vi "Dresden R2R Sputter 03.02.2018 IY24.vi"() -> ()   [LabVIEW 2009] (continued)
                                n27365 = local read "R Single DC Interval length"() -> (w32478:dbl)
                                n27366 = local read "Actual Length"() -> (w32482:dbl)
                                n27367 = Multiply(x=w32478, y=5.0) -> (x*y=w32476:dbl)
                                n27368 = Greater Or Equal?(x=w32482, y=w32476) -> (x >= y?=w32481:bool)
                                n27369 = local read "Semi"() -> (w32480:bool)
                                n27370 = Or(x=w32481, y=w32480) -> (x .or. y?=w32479:bool)
                                n27371 = Wait Until Next ms Multiple(millisecond multiple=u32 300) -> ()  [unwired: 1 out]
                                }
                                }
                                }
                                }
                                }
                                }
                                }
                                }
                                frame #1 {
                                }
                                }
                                }
                                frame #13 {
                                n27372 = local read "Semi"() -> (w32483:bool)
                                n27373 = case shown="False" w32483 {
                                frame #0 {
                                n27374 = local write "SDC1 13b"(TRUE ("SDC1 13b")) -> ()
                                n27375 = Wait (ms)(milliseconds to wait=u32 1000) -> ()  [unwired: 1 out]
                                }
                                frame #1 {
                                }
                                }
                                }
                                }
                                }
                                frame #1 {
                                }
                                }
                                }
                                frame #17 {
                                # "encoder info  add to other web selection"
                                n27376 = stacked-sequence {
                                frame #0 {
                                n27377 = local read "Semi"() -> (w32486:bool)
                                n27378 = case shown="False" w32486 {
                                frame #0 {
                                # "salinim hareketi"
                                n27379 = local read "R_Web_selection"() -> (w32487:enum32{"Web", "Other"})
                                n27380 = case shown="\"Other\"" w32487 {
                                frame #0 {
                                # "TC -ROLL"
                                }
                                frame #1 {
                                n27381 = disable-structure shown="Disabled" {
                                frame #0 {
                                # "OTHER"
                                n27382 = local read "Semi"() -> (w32488:bool)
                                n27383 = case shown="False" w32488 {
                                frame #0 {
                                n27384 = stacked-sequence {
                                frame #0 {
                                n27385 = local read "Semi"() -> (w32489:bool)
                                n27386 = case shown="False" w32489 {
                                frame #0 {
                                n27387 = stacked-sequence {
                                frame #0 {
                                n27388 = local read "Semi"() -> (w32490:bool)
                                n27389 = case shown="False" w32490 {
                                frame #0 {
                                n27390 = while {
                                i -> [w32493]
                                stop <- w32494 stop-if-true
                                n27391 = Greater?(x=w32493, y=300) -> (0:w32491:bool)
                                n27392 = case shown="True" w32491 {
                                frame #0 {
                                }
                                frame #1 {
                                n27393 = local write "Semi"(TRUE ("Semi")) -> ()
                                }
                                }
                                n27394 = local read "RC_13"() -> (w32497:bool)
                                n27395 = case shown="False" w32497 {
                                tunnel: [FALSE ("ch2_1") TRUE ("ch2_1")] -> w32496
                                frame #0 {
                                n27396 = local write "Routine_check_transfer"(TRUE ("ch2_1")) -> ()
                                n27397 = Wait Until Next ms Multiple(millisecond multiple=u32 1000) -> ()  [unwired: 1 out]
                                }
                                frame #1 {
                                }
                                }
                                n27398 = local read "Semi"() -> (w32495:bool)
                                n27399 = Or(x=w32496, y=w32495) -> (x .or. y?=w32494:bool)
                                }
                                }
                                frame #1 {
                                }
                                }
                                }
                                frame #1 {
                                n27400 = local read "Semi"() -> (w32503:bool)
                                n27401 = case shown="False" w32503 {
                                frame #0 {
                                n27402 = while {
                                i -> [w32510]
                                stop <- w32505 stop-if-true
                                n27403 = Greater?(x=w32510, y=100) -> (0:w32508:bool)
                                n27404 = case shown="True" w32508 {
                                frame #0 {
                                }
                                frame #1 {
                                n27405 = local write "Error Message"("Transfer process was cancelled.\nPlease check GV connections." ("Error Message")) -> ()
                                n27406 = local write "Semi"(TRUE ("Semi")) -> ()
                                }
                                }
                                n27407 = local read "Ch1_Trns_interlock_di"() -> (w32504:bool)
                                n27408 = case shown="False" w32504 {
                                tunnel: [w32512 TRUE] -> w32507
                                frame #0 {
                                n27409 = local read "Ch1_TGV_control_di"() -> (w32511:bool)
                                n27410 = case shown="False" w32511 {
                                tunnel: [FALSE TRUE] -> w32512
                                frame #0 {
                                n27411 = Wait Until Next ms Multiple(millisecond multiple=u32 50) -> ()  [unwired: 1 out]
                                n27412 = local write "Ch1_TGV_control_do"(TRUE ("Ch1_pet_cool_up_do")) -> ()
                                }
                                frame #1 {
                                }
                                }
                                }
                                frame #1 {
                                }
                                }
                                n27413 = local read "Semi"() -> (w32506:bool)
                                n27414 = Or(x=w32507, y=w32506) -> (x .or. y?=w32505:bool)
                                }
                                }
                                frame #1 {
                                }
                                }
                                }
                                frame #2 {
                                n27415 = local read "Semi"() -> (w32520:bool)
                                n27416 = case shown="False" w32520 {
                                frame #0 {
                                n27417 = while {
                                i -> [w32527]
                                stop <- w32522 stop-if-true
                                n27418 = Greater?(x=w32527, y=100) -> (0:w32525:bool)
                                n27419 = case shown="True" w32525 {
                                frame #0 {
                                }
                                frame #1 {
                                n27420 = local write "Error Message"("Transfer process was cancelled.\nPlease check GV connections." ("Error Message")) -> ()
                                n27421 = local write "Semi"(TRUE ("Semi")) -> ()
                                }
                                }
                                n27422 = local read "Ch2_Trns_interlock_di"() -> (w32521:bool)
                                n27423 = case shown="False" w32521 {
                                tunnel: [w32529 TRUE] -> w32524
                                frame #0 {
                                n27424 = local read "Ch2_TGV_control_di"() -> (w32528:bool)
                                n27425 = case shown="False" w32528 {
                                tunnel: [FALSE TRUE] -> w32529
                                frame #0 {
                                n27426 = Wait Until Next ms Multiple(millisecond multiple=u32 50) -> ()  [unwired: 1 out]
                                n27427 = local write "Ch2_TGV_control_do"(TRUE ("Ch1_pet_cool_up_do")) -> ()
                                }
                                frame #1 {
                                }
                                }
                                }
                                frame #1 {
                                }
                                }
                                n27428 = local read "Semi"() -> (w32523:bool)
                                n27429 = Or(x=w32524, y=w32523) -> (x .or. y?=w32522:bool)
                                }
                                }
                                frame #1 {
                                }
                                }
                                }
                                frame #3 {
                                n27430 = local read "Semi"() -> (w32537:bool)
                                n27431 = case shown="False" w32537 {
                                frame #0 {
                                n27432 = while {
                                i -> [w32544]
                                stop <- w32539 stop-if-true
                                n27433 = Greater?(x=w32544, y=100) -> (0:w32542:bool)
                                n27434 = case shown="True" w32542 {
                                frame #0 {
                                }
                                frame #1 {
                                n27435 = local write "Error Message"("Transfer process was cancelled.\nPlease check GV connections." ("Error Message")) -> ()
                                n27436 = local write "Semi"(TRUE ("Semi")) -> ()
                                }
                                }
                                n27437 = local read "Ch3_Trns_interlock_di"() -> (w32538:bool)
                                n27438 = case shown="False" w32538 {
                                tunnel: [w32546 TRUE] -> w32541
                                frame #0 {
                                n27439 = local read "Ch3_TGV_control_di"() -> (w32545:bool)
                                n27440 = case shown="False" w32545 {
                                tunnel: [FALSE TRUE] -> w32546
                                frame #0 {
                                n27441 = Wait Until Next ms Multiple(millisecond multiple=u32 50) -> ()  [unwired: 1 out]
                                n27442 = local write "Ch3_TGV_control_do"(TRUE ("Ch1_pet_cool_up_do")) -> ()
                                }
                                frame #1 {
                                }
                                }
                                }
                                frame #1 {
                                }
                                }
                                n27443 = local read "Semi"() -> (w32540:bool)
                                n27444 = Or(x=w32541, y=w32540) -> (x .or. y?=w32539:bool)
                                }
                                }
                                frame #1 {
                                }
                                }
                                }
                                frame #4 {
                                n27445 = local read "Semi"() -> (w32554:bool)
                                n27446 = case shown="False" w32554 {
                                frame #0 {
                                n27447 = while {
                                i -> [w32561]
                                stop <- w32556 stop-if-true
                                n27448 = Greater?(x=w32561, y=100) -> (0:w32559:bool)
                                n27449 = case shown="True" w32559 {
                                frame #0 {
                                }
                                frame #1 {
                                n27450 = local write "Error Message"("Transfer process was cancelled.\nPlease check GV connections." ("Error Message")) -> ()
                                n27451 = local write "Semi"(TRUE ("Semi")) -> ()
                                }
                                }
                                n27452 = local read "Ch3_Trns_interlock_di"() -> (w32555:bool)
                                n27453 = case shown="False" w32555 {
                                tunnel: [w32563 TRUE] -> w32558
                                frame #0 {
                                n27454 = local read "Ch3_TGV_control_di"() -> (w32562:bool)
                                n27455 = case shown="False" w32562 {
                                tunnel: [FALSE TRUE] -> w32563
                                frame #0 {
                                n27456 = Wait Until Next ms Multiple(millisecond multiple=u32 50) -> ()  [unwired: 1 out]
                                n27457 = local write "Ch3_TGV_control_do"(TRUE ("Ch1_pet_cool_up_do")) -> ()
                                }
                                frame #1 {
                                }
                                }
                                }
                                frame #1 {
                                }
                                }
                                n27458 = local read "Semi"() -> (w32557:bool)
                                n27459 = Or(x=w32558, y=w32557) -> (x .or. y?=w32556:bool)
                                }
                                }
                                frame #1 {
                                }
                                }
                                }
                                frame #5 {
                                n27460 = local read "Semi"() -> (w32571:bool)
                                n27461 = case shown="False" w32571 {
                                frame #0 {
                                n27462 = while {
                                i -> [w32574]
                                stop <- w32575 stop-if-true
                                n27463 = Greater?(x=w32574, y=50) -> (0:w32572:bool)
                                n27464 = case shown="True" w32572 {
                                frame #0 {
                                }
                                frame #1 {
                                n27465 = local write "Error Message"("Transfer process was\ncancelled.Please check right slow sensor." ("Error Message")) -> ()
                                n27466 = local write "Semi"(TRUE ("Semi")) -> ()
                                }
                                }
                                n27467 = local read "Cnt_Right_slow_di"() -> (w32578:bool)
                                n27468 = case shown="False" w32578 {
                                tunnel: [FALSE ("Ch1_pet_cool_up_do") TRUE ("Ch1_pet_cool_up_do")] -> w32577
                                frame #0 {
                                n27469 = local write "Cnt_Right_slow_do"(TRUE ("Ch1_pet_cool_up_do")) -> ()
                                n27470 = Wait Until Next ms Multiple(millisecond multiple=u32 200) -> ()  [unwired: 1 out]
                                }
                                frame #1 {
                                }
                                }
                                n27471 = local read "Semi"() -> (w32576:bool)
                                n27472 = Or(x=w32577, y=w32576) -> (x .or. y?=w32575:bool)
                                }
                                }
                                frame #1 {
                                }
                                }
                                }
                                frame #6 {
                                n27473 = local read "Semi"() -> (w32585:bool)
                                n27474 = case shown="False" w32585 {
                                frame #0 {
                                n27475 = while {
                                i -> [w32586]
                                stop <- w32590 stop-if-true
                                n27476 = Greater?(x=w32586, y=50) -> (0:w32588:bool)
                                n27477 = case shown="True" w32588 {
                                frame #0 {
                                }
                                frame #1 {
                                n27478 = local write "Error Message"("Transfer process was\ncancelled.Please check right limit sensor." ("Error Message")) -> ()
                                n27479 = local write "Semi"(TRUE ("Semi")) -> ()
                                }
                                }
                                n27480 = local read "Cnt_Right_limit_di"() -> (w32592:bool)
                                n27481 = case shown="False" w32592 {
                                tunnel: [FALSE ("Ch1_pet_cool_up_do") TRUE ("Ch1_pet_cool_up_do")] -> w32591
                                frame #0 {
                                n27482 = local write "Cnt_Right_limit_do"(TRUE ("Ch1_pet_cool_up_do")) -> ()
                                n27483 = Wait Until Next ms Multiple(millisecond multiple=u32 200) -> ()  [unwired: 1 out]
                                }
                                frame #1 {
                                }
                                }
                                n27484 = local read "Semi"() -> (w32589:bool)
                                n27485 = Or(x=w32591, y=w32589) -> (x .or. y?=w32590:bool)
                                }
                                }
                                frame #1 {
                                }
                                }
                                }
                                frame #7 {
                                n27486 = local read "Semi"() -> (w32599:bool)
                                n27487 = case shown="False" w32599 {
                                frame #0 {
                                n27488 = while {
                                i -> [w32602]
                                stop <- w32603 stop-if-true
                                n27489 = Greater?(x=w32602, y=50) -> (0:w32600:bool)
                                n27490 = case shown="True" w32600 {
                                frame #0 {
                                }
                                frame #1 {
                                n27491 = local write "Error Message"("Transfer process was\ncancelled.Please check left slow sensor." ("Error Message")) -> ()
                                n27492 = local write "Semi"(TRUE ("Semi")) -> ()
                                }
                                }
                                n27493 = local read "Cnt_Left_slow_di"() -> (w32606:bool)
                                n27494 = case shown="False" w32606 {
                                tunnel: [FALSE ("Ch1_pet_cool_up_do") TRUE ("Ch1_pet_cool_up_do")] -> w32605
                                frame #0 {
                                n27495 = local write "Cnt_Left_slow_do"(TRUE ("Ch1_pet_cool_up_do")) -> ()
                                n27496 = Wait Until Next ms Multiple(millisecond multiple=u32 200) -> ()  [unwired: 1 out]
                                }
                                frame #1 {
                                }
                                }
                                n27497 = local read "Semi"() -> (w32604:bool)
                                n27498 = Or(x=w32605, y=w32604) -> (x .or. y?=w32603:bool)
                                }
                                }
                                frame #1 {
                                }
                                }
                                }
                                frame #8 {
                                n27499 = local read "Semi"() -> (w32613:bool)
                                n27500 = case shown="False" w32613 {
                                frame #0 {
                                n27501 = while {
                                i -> [w32614]
                                stop <- w32618 stop-if-true
                                n27502 = Greater?(x=w32614, y=50) -> (0:w32616:bool)
                                n27503 = case shown="True" w32616 {
                                frame #0 {
                                }
                                frame #1 {
                                n27504 = local write "Error Message"("Transfer process was\ncancelled.Please check left limit sensor." ("Error Message")) -> ()
                                n27505 = local write "Semi"(TRUE ("Semi")) -> ()
                                }
                                }
                                n27506 = local read "Cnt_Left_limit_di"() -> (w32620:bool)
                                n27507 = case shown="False" w32620 {
                                tunnel: [FALSE ("Ch1_pet_cool_up_do") TRUE ("Ch1_pet_cool_up_do")] -> w32619
                                frame #0 {
                                n27508 = local write "Cnt_Left_limit_do"(TRUE ("Ch1_pet_cool_up_do")) -> ()
                                n27509 = Wait Until Next ms Multiple(millisecond multiple=u32 200) -> ()  [unwired: 1 out]
                                }
                                frame #1 {
                                }
                                }
                                n27510 = local read "Semi"() -> (w32617:bool)
                                n27511 = Or(x=w32619, y=w32617) -> (x .or. y?=w32618:bool)
                                }
                                }
                                frame #1 {
                                }
                                }
                                }
                                }
                                }
                                frame #1 {
                                }
                                }
                                }
                                frame #1 {
                                n27512 = local read "Semi"() -> (w32627:bool)
                                n27513 = case shown="False" w32627 {
                                frame #0 {
                                n27514 = while {
                                i -> [w32633]
                                stop <- w32630 stop-if-true
                                n27515 = Greater?(x=w32633, y=50) -> (0:w32632:bool)
                                n27516 = case shown="True" w32632 {
                                frame #0 {
                                }
                                frame #1 {
                                n27517 = local write "Error Message"("" ("Error Message")) -> ()
                                n27518 = local write "Semi"(TRUE ("Semi")) -> ()
                                }
                                }
                                n27519 = local read "Casette_servo_start/stop_di"() -> (w32629:bool)
                                n27520 = case shown="False" w32629 {
                                tunnel: [FALSE TRUE] -> w32628
                                frame #0 {
                                n27521 = local write "Casette_servo_start/stop_do"(TRUE ("Casette_servo_left_direction_do")) -> ()
                                n27522 = Wait Until Next ms Multiple(millisecond multiple=u32 500) -> ()  [unwired: 1 out]
                                }
                                frame #1 {
                                }
                                }
                                n27523 = local read "Semi"() -> (w32631:bool)
                                n27524 = Or(x=w32628, y=w32631) -> (x .or. y?=w32630:bool)
                                }
                                }
                                frame #1 {
                                }
                                }
                                }
                                frame #2 {
                                n27525 = local read "Semi"() -> (w32641:bool)
                                n27526 = case shown="False" w32641 {
                                frame #0 {
                                n27527 = while {
                                i -> [w32647]
                                stop <- w32644 stop-if-true
                                n27528 = Greater?(x=w32647, y=50) -> (0:w32646:bool)
                                n27529 = case shown="True" w32646 {
                                frame #0 {
                                }
                                frame #1 {
                                n27530 = local write "Error Message"("" ("Error Message")) -> ()
                                n27531 = local write "Semi"(TRUE ("Semi")) -> ()
                                }
                                }
                                n27532 = local read "Casette_servo_left_direction_di"() -> (w32643:bool)
                                n27533 = case shown="False" w32643 {
                                tunnel: [FALSE TRUE] -> w32642
                                frame #0 {
                                n27534 = local write "Casette_servo_left_direction_do"(TRUE ("Casette_servo_left_direction_do")) -> ()
                                n27535 = Wait Until Next ms Multiple(millisecond multiple=u32 200) -> ()  [unwired: 1 out]
                                }
                                frame #1 {
                                }
                                }
                                n27536 = local read "Semi"() -> (w32645:bool)
                                n27537 = Or(x=w32642, y=w32645) -> (x .or. y?=w32644:bool)
                                }
                                }
                                frame #1 {
                                }
                                }
                                }
                                frame #3 {
                                # "casette motion"
                                n27538 = while {
                                i -> [w32657]
                                stop <- w32655 stop-if-true
                                n27539 = Greater?(x=w32657, y=200) -> (0:w32658:bool)
                                n27540 = case shown="True" w32658 {
                                frame #0 {
                                }
                                frame #1 {
                                n27541 = local write "Semi"(TRUE ("Semi")) -> ()
                                }
                                }
                                n27542 = local read "Counter_read_data"() -> (w32663:i16)
                                n27543 = Greater?(x=w32663, y=i16 0) -> (0:w32661:bool)
                                n27544 = case shown="True" w32661 {
                                tunnel: [TRUE TRUE] -> w32660
                                frame #0 {
                                }
                                frame #1 {
                                n27545 = local write "Casette_servo_start/stop_do"(FALSE ("Casette_servo_start/stop_do")) -> ()
                                n27546 = Wait Until Next ms Multiple(millisecond multiple=u32 200) -> ()  [unwired: 1 out]
                                }
                                }
                                n27547 = local read "Semi"() -> (w32659:bool)
                                n27548 = Or(x=w32660, y=w32659) -> (x .or. y?=w32655:bool)
                                }
                                }
                                frame #4 {
                                n27549 = local read "Semi"() -> (w32669:bool)
                                n27550 = case shown="False" w32669 {
                                frame #0 {
                                n27551 = while {
                                i -> [w32675]
                                stop <- w32672 stop-if-true
                                n27552 = Greater?(x=w32675, y=50) -> (0:w32674:bool)
                                n27553 = case shown="True" w32674 {
                                frame #0 {
                                }
                                frame #1 {
                                n27554 = local write "Error Message"("" ("Error Message")) -> ()
                                n27555 = local write "Semi"(TRUE ("Semi")) -> ()
                                }
                                }
                                n27556 = local read "Casette_servo_start/stop_di"() -> (w32671:bool)
                                n27557 = case shown="True" w32671 {
                                tunnel: [TRUE FALSE] -> w32670
                                frame #0 {
                                }
                                frame #1 {
                                n27558 = local write "Casette_servo_start/stop_do"(FALSE ("Casette_servo_left_direction_do")) -> ()
                                n27559 = Wait Until Next ms Multiple(millisecond multiple=u32 500) -> ()  [unwired: 1 out]
                                }
                                }
                                n27560 = local read "Semi"() -> (w32673:bool)
                                n27561 = Or(x=w32670, y=w32673) -> (x .or. y?=w32672:bool)
                                }
                                }
                                frame #1 {
                                }
                                }
                                }
                                frame #5 {
                                n27562 = local read "Semi"() -> (w32683:bool)
                                n27563 = case shown="False" w32683 {
                                frame #0 {
                                n27564 = Wait (ms)(milliseconds to wait=u32 5000 ("millisecond multiple 4")) -> ()  [unwired: 1 out]
                                }
                                frame #1 {
                                }
                                }
                                }
                                frame #6 {
                                n27565 = local read "Semi"() -> (w32685:bool)
                                n27566 = case shown="False" w32685 {
                                frame #0 {
                                n27567 = while {
                                i -> [w32691]
                                stop <- w32688 stop-if-true
                                n27568 = Greater?(x=w32691, y=50) -> (0:w32690:bool)
                                n27569 = case shown="True" w32690 {
                                frame #0 {
                                }
                                frame #1 {
                                n27570 = local write "Error Message"("" ("Error Message")) -> ()
                                n27571 = local write "Semi"(TRUE ("Semi")) -> ()
                                }
                                }
                                n27572 = local read "Casette_servo_start/stop_di"() -> (w32687:bool)
                                n27573 = case shown="False" w32687 {
                                tunnel: [FALSE TRUE] -> w32686
                                frame #0 {
                                n27574 = local write "Casette_servo_start/stop_do"(TRUE ("Casette_servo_left_direction_do")) -> ()
                                n27575 = Wait Until Next ms Multiple(millisecond multiple=u32 500) -> ()  [unwired: 1 out]
                                }
                                frame #1 {
                                }
                                }
                                n27576 = local read "Semi"() -> (w32689:bool)
                                n27577 = Or(x=w32686, y=w32689) -> (x .or. y?=w32688:bool)
                                }
                                }
                                frame #1 {
                                }
                                }
                                }
                                frame #7 {
                                n27578 = local read "Semi"() -> (w32699:bool)
                                n27579 = case shown="False" w32699 {
                                frame #0 {
                                n27580 = while {
                                i -> [w32705]
                                stop <- w32702 stop-if-true
                                n27581 = Greater?(x=w32705, y=50) -> (0:w32704:bool)
                                n27582 = case shown="True" w32704 {
                                frame #0 {
                                }
                                frame #1 {
                                n27583 = local write "Error Message"("" ("Error Message")) -> ()
                                n27584 = local write "Semi"(TRUE ("Semi")) -> ()
                                }
                                }
                                n27585 = local read "Casette_servo_left_direction_di"() -> (w32701:bool)
                                n27586 = case shown="True" w32701 {
                                tunnel: [TRUE FALSE] -> w32700
                                frame #0 {
                                }
                                frame #1 {
                                n27587 = local write "Casette_servo_left_direction_do"(FALSE ("Casette_servo_left_direction_do")) -> ()
                                n27588 = Wait Until Next ms Multiple(millisecond multiple=u32 200) -> ()  [unwired: 1 out]
                                }
                                }
                                n27589 = local read "Semi"() -> (w32703:bool)
                                n27590 = Or(x=w32700, y=w32703) -> (x .or. y?=w32702:bool)
                                }
                                }
                                frame #1 {
                                }
                                }
                                }
                                frame #8 {
                                # "casette motion"
                                n27591 = while {
                                i -> [w32716]
                                stop <- w32713 stop-if-true
                                n27592 = Greater?(x=w32716, y=200) -> (0:w32717:bool)
                                n27593 = case shown="True" w32717 {
                                frame #0 {
                                }
                                frame #1 {
                                n27594 = local write "Semi"(TRUE ("Semi")) -> ()
                                }
                                }
                                n27595 = local read "Counter_read_data"() -> (w32721:i16)
                                n27596 = Less?(x=w32721, y=i16 0) -> (x < y?=w32720:bool)
                                n27597 = case shown="True" w32720 {
                                tunnel: [TRUE TRUE] -> w32719
                                frame #0 {
                                }
                                frame #1 {
                                n27598 = local write "Casette_servo_start/stop_do"(FALSE ("Casette_servo_start/stop_do")) -> ()
                                n27599 = Wait Until Next ms Multiple(millisecond multiple=u32 200) -> ()  [unwired: 1 out]
                                }
                                }
                                n27600 = local read "Semi"() -> (w32718:bool)
                                n27601 = Or(x=w32719, y=w32718) -> (x .or. y?=w32713:bool)
                                }
                                }
                                frame #9 {
                                n27602 = local read "Semi"() -> (w32727:bool)
                                n27603 = case shown="False" w32727 {
                                frame #0 {
                                n27604 = while {
                                i -> [w32733]
                                stop <- w32730 stop-if-true
                                n27605 = Greater?(x=w32733, y=50) -> (0:w32732:bool)
                                n27606 = case shown="True" w32732 {
                                frame #0 {
                                }
                                frame #1 {
                                n27607 = local write "Error Message"("" ("Error Message")) -> ()
                                n27608 = local write "Semi"(TRUE ("Semi")) -> ()
                                }
                                }
                                n27609 = local read "Casette_servo_start/stop_di"() -> (w32729:bool)
                                n27610 = case shown="True" w32729 {
                                tunnel: [TRUE FALSE] -> w32728
                                frame #0 {
                                }
                                frame #1 {
                                n27611 = local write "Casette_servo_start/stop_do"(FALSE ("Casette_servo_left_direction_do")) -> ()
                                n27612 = Wait Until Next ms Multiple(millisecond multiple=u32 500) -> ()  [unwired: 1 out]
                                }
                                }
                                n27613 = local read "Semi"() -> (w32731:bool)
                                n27614 = Or(x=w32728, y=w32731) -> (x .or. y?=w32730:bool)
                                }
                                }
                                frame #1 {
                                }
                                }
                                }
                                frame #10 {
                                n27615 = local read "Semi"() -> (w32741:bool)
                                n27616 = case shown="False" w32741 {
                                frame #0 {
                                n27617 = local write "SDC1 21b"(TRUE ("SDC1 21b")) -> ()
                                }
                                frame #1 {
                                }
                                }
                                }
                                }
                                }
                                frame #1 {
                                }
                                }
                                }
                                frame #1 {
                                }
                                }
                                }
                                }
                                }
                                frame #1 {
                                }
                                }
                                }
                                frame #1 {
                                n27618 = local read "Semi"() -> (w32743:bool)
                                n27619 = case shown="False" w32743 {
                                frame #0 {
                                n27620 = Wait (ms)(milliseconds to wait=u32 1000) -> ()  [unwired: 1 out]
                                n27621 = local write "SDC1 21"(TRUE ("SDC1 21")) -> ()
                                }
                                frame #1 {
                                }
                                }
                                }
                                }
                                }
                                frame #18 {
                                # "tm parameter"
                                n27622 = local read "Semi"() -> (w32746:bool)
                                n27623 = case shown="False" w32746 {
                                frame #0 {
                                n27624 = local read "Thickness_Monitor_Active"() -> (w32747:bool)
                                n27625 = case shown="True" w32747 {
                                frame #0 {
                                }
                                frame #1 {
                                n27626 = local read "Semi"() -> (w32748:bool)
                                n27627 = case shown="False" w32748 {
                                frame #0 {
                                n27628 = stacked-sequence {
                                frame #0 {
                                n27629 = local read "Semi"() -> (w32749:bool)
                                n27630 = case shown="False" w32749 {
                                frame #0 {
                                n27631 = local read "R Toooling_factor"() -> (w32750:dbl)
                                n27632 = local read "R Material_density"() -> (w32752:dbl)
                                n27633 = local read "R Z_factor"() -> (w32751:dbl)
                                n27634 = local write "Tooling_factor2"(w32750) -> ()
                                n27635 = local write "Material_density2"(w32752) -> ()
                                n27636 = local write "Z_factor2"(w32751) -> ()
                                }
                                frame #1 {
                                }
                                }
                                }
                                frame #1 {
                                n27637 = local read "Semi"() -> (w32753:bool)
                                n27638 = case shown="False" w32753 {
                                frame #0 {
                                n27639 = Wait (ms)(milliseconds to wait=u32 1000) -> ()  [unwired: 1 out]
                                }
                                frame #1 {
                                }
                                }
                                }
                                frame #2 {
                                n27640 = local read "Semi"() -> (w32755:bool)
                                n27641 = case shown="False" w32755 {
                                frame #0 {
                                n27642 = local read "R Single DC Target material"() -> (w32756:string)
                                n27643 = Write to Text File(file (use dialog)=path path "D/VK-1701 System Files/Material Data/data2.txt", text=w32756) -> ()  [unwired: 2 in, 3 out]
                                }
                                frame #1 {
                                }
                                }
                                }
                                frame #3 {
                                n27644 = local read "Semi"() -> (w32758:bool)
                                n27645 = case shown="False" w32758 {
                                frame #0 {
                                n27646 = local write "SDC1 22"(TRUE ("SDC1 22")) -> ()
                                n27647 = Wait (ms)(milliseconds to wait=u32 1000) -> ()  [unwired: 1 out]
                                }
                                frame #1 {
                                }
                                }
                                }
                                }
                                }
                                frame #1 {
                                }
                                }
                                }
                                }
                                }
                                frame #1 {
                                }
                                }
                                }
                                frame #19 {
                                n27648 = local read "Semi"() -> (w32761:bool)
                                n27649 = case shown="False" w32761 {
                                frame #0 {
                                n27650 = local read "R_Web_selection"() -> (w32762:enum32{"Web", "Other"})
                                n27651 = case shown="\"Other\"" w32762 {